vi "Show_Queued_Images.vi"(8 "error in (no error)":errorcluster, 11 "ImagesQueue":string) -> (0 "error out":errorcluster)   [LabVIEW 2016]
uses:
  <vilib>/vision/Image Controls.llb/IMAQ Image.ctl
panel:
  out "Image":T1(plugin-control)
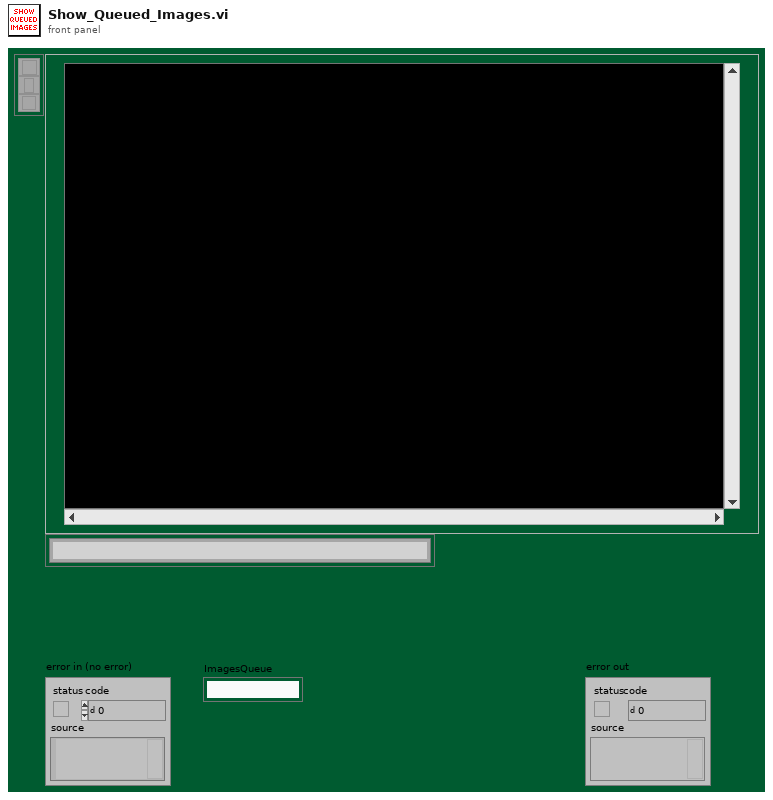
[diagram p1: front panel]
types:
  T1 = typedef "IMAQ Image.ctl" = refnum<image>
  T2 = enum16{"Show:ResetError", "Show:Exit", "Show:QueueError", "Show;Timeout_Image_Queue", "Show:Error_Imaq", "Show:Reset_Error_Recvd"}
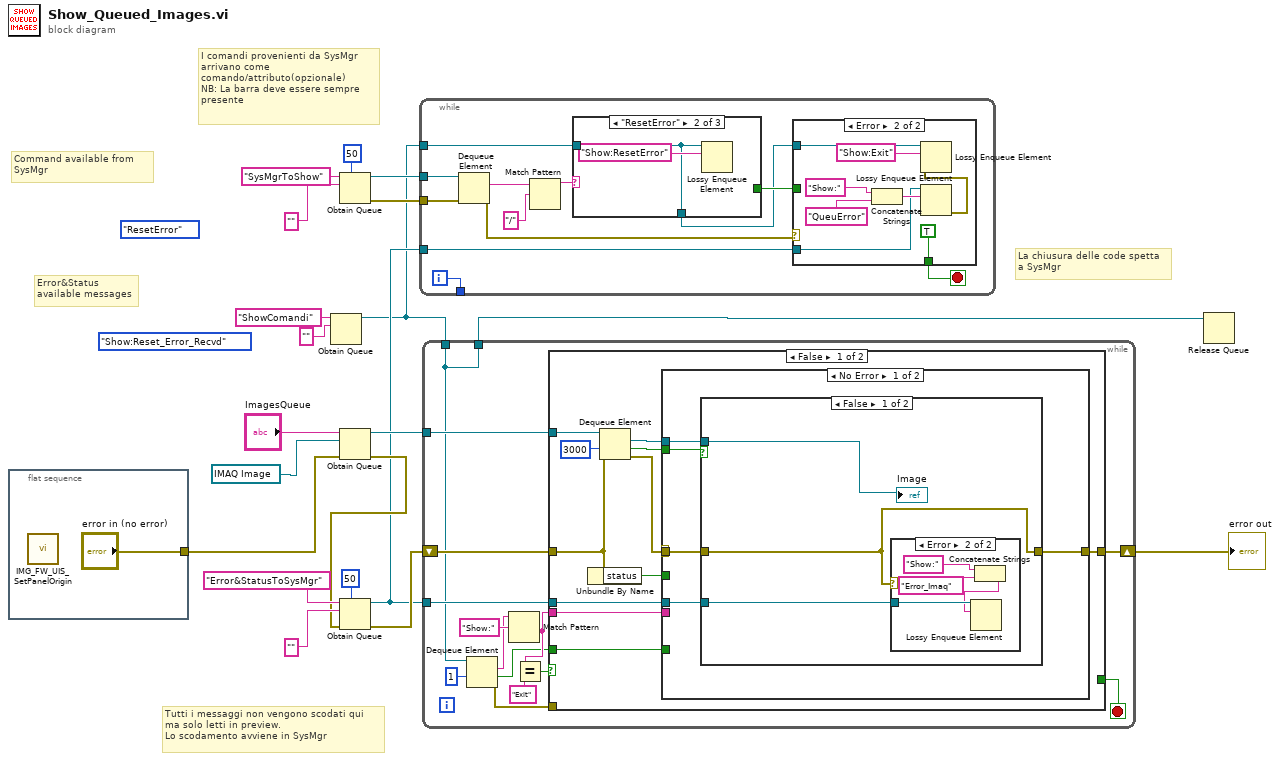
[diagram p0: block diagram]
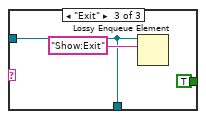
[diagram p4: hidden frame]
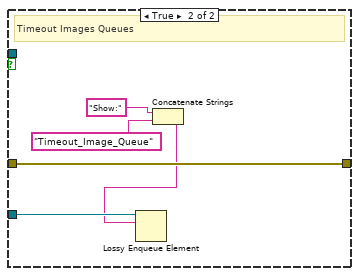
[diagram p6: hidden frame]
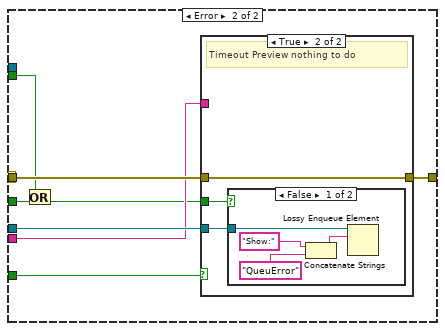
[diagram p7: hidden frame]
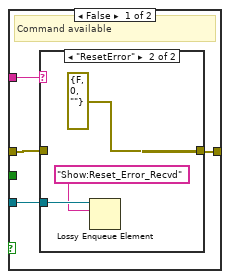
[diagram p8: hidden frame]
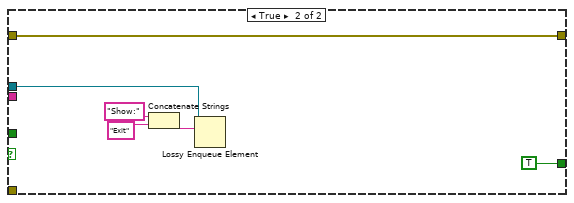
[diagram p11: hidden frame]
diagram:
  (unwired) T2."Show:Reset_Error_Recvd"
  (unwired) enum16{"Exit", "ResetError"}."ResetError"
  # "Tutti i messaggi non vengono scodati qui\nma solo letti in preview.\nLo scodamento avviene in SysMgr"
  # "Error&Status\navailable messages"
  # "Command available from \nSysMgr"
  # "La chiusura delle code spetta\na SysMgr"
  # "I comandi provenienti da SysMgr \narrivano come\ncomando/attributo(opzionale)\nNB: La barra deve essere sempre \npresente"
  n1 = flat-sequence {
    tunnel: ["error in (no error)"] -> w9
    frame #0 {
      n2 = call "IMG_FW_UIS_SetPanelOrigin.vi"() -> ()  [unwired: 11 in, 1 out]
    }
  }
  n3 = Obtain Queue(name (unnamed)="ShowComandi", element data type="") -> (queue out=w3:refnum<queue>)  [unwired: 3 in, 2 out]
  n4 = Obtain Queue(max queue size (-1, unlimited)=50, name (unnamed)="SysMgrToShow", element data type="") -> (queue out=w16:refnum<queue>, error out=w10:errorcluster)  [unwired: 2 in, 1 out]
  n5 = Obtain Queue(name (unnamed)="ImagesQueue", element data type=T1 refnum ("Image"), error in (no error)=w9) -> (queue out=w19:refnum<queue>, error out=w8:errorcluster)  [unwired: 2 in, 1 out]
  n6 = Obtain Queue(max queue size (-1, unlimited)=50, name (unnamed)="Error&StatusToSysMgr", element data type="", error in (no error)=w8) -> (queue out=w4:refnum<queue>, error out=w7:errorcluster)  [unwired: 1 in, 1 out]
  n7 = while {
    tunnel: w16 -> [w33]
    tunnel: w10 -> [w29]
    tunnel: w4 -> [w26]
    tunnel: [w24] -> _
    tunnel: w3 -> [w22]
    i -> [w24]
    stop <- w27 stop-if-true
    n8 = Dequeue Element(queue=w33, error in (no error)=w29) -> (element=w32:string, error out=w28:errorcluster)  [unwired: 1 in, 2 out]
    n9 = Match Pattern(string=w32, regular expression="/") -> (before substring=w30:string)  [unwired: 1 in, 3 out]
    n10 = case shown="\"ResetError\"" w30 {
      tunnel: [w43 w44 w46] -> w23
      tunnel: [_ _ TRUE] -> w25
      tunnel: w22 -> [w43 w44 w46]
      frame "", Default {
      }
      frame "ResetError" {
        n11 = Lossy Enqueue Element(queue=w44, element="Show:ResetError" ("notification")) -> ()  [unwired: 1 in, 4 out]
      }
      frame "Exit" {
        n12 = Lossy Enqueue Element(queue=w46, element="Show:Exit" ("notification")) -> ()  [unwired: 1 in, 4 out]
      }
    }
    n13 = case shown="Error" w28 {
      tunnel: [w34 TRUE] -> w27
      tunnel: w26 -> [_ w38]
      tunnel: w25 -> [w34 _]
      tunnel: w23 -> [_ w35]
      frame No Error {
      }
      frame Error {
        n14 = Concatenate Strings("Show:", "QueuError") -> (w39:string)
        n15 = Lossy Enqueue Element(queue=w38, element=w39) -> (error out=w37:errorcluster)  [unwired: 1 in, 3 out]
        n16 = Lossy Enqueue Element(queue=w35, element="Show:Exit" ("notification"), error in (no error)=w37) -> ()  [unwired: 4 out]
      }
    }
  }
  n17 = while {
    tunnel: w19 -> [w62]
    tunnel: w4 -> [w56]
    shift-right: [w61] -> w18
    shift-left: w7 -> [w60]
    tunnel: w3 -> [w52]
    tunnel: [w52] -> w2
    stop <- w54 stop-if-true
    n18 = Dequeue Element(queue=w52, timeout in ms (-1)=1) -> (element=w51:string, timed out?=w49:bool, error out=w53:errorcluster)  [unwired: 1 in, 1 out]
    n19 = Match Pattern(string=w51, regular expression="Show:") -> (after substring=w50:string)  [unwired: 1 in, 3 out]
    n20 = Equal?(x=w50, y="Exit") -> (x = y?=w55:bool)
    n21 = case shown="False" w55 {
      tunnel: w62 -> [w73 _]
      tunnel: [w71 w119] -> w61
      tunnel: w60 -> [w67 w119]
      tunnel: w56 -> [w65 w115]
      tunnel: [_ TRUE] -> w54
      tunnel: w53 -> [_ _]
      tunnel: w50 -> [w64 _]
      tunnel: w49 -> [w63 _]
      frame False {
        n22 = Unbundle By Name(w67) -> ("status"=w66:bool)
        n23 = Dequeue Element(queue=w73, timeout in ms (-1)=3000, error in (no error)=w67) -> (element=w72:T1, timed out?=w69:bool, error out=w68:errorcluster)  [unwired: 1 out]
        n24 = case shown="No Error" w68 {
          selector: w68 -> [w75 w98]
          tunnel: w72 -> [w78 _]
          tunnel: w68 -> [_ _]
          tunnel: [w77 w97] -> w71
          tunnel: w69 -> [w76 w94]
          tunnel: w65 -> [w74 w96]
          tunnel: w66 -> [_ w95]
          tunnel: w64 -> [_ w93]
          tunnel: w63 -> [_ w91]
          frame No Error {
            n25 = case shown="False" w76 {
              tunnel: w78 -> [w80 _]
              tunnel: w75 -> [w79 w90]
              tunnel: [w79 w90] -> w77
              tunnel: w74 -> [w81 w89]
              frame False {
                n26 = case shown="Error" w79 {
                  tunnel: w81 -> [_ w85]
                  frame No Error {
                  }
                  frame Error {
                    n27 = Concatenate Strings("Show:", "Error_Imaq") -> (w83:string)
                    n28 = Lossy Enqueue Element(queue=w85, element=w83) -> ()  [unwired: 1 in, 4 out]
                  }
                }
                "Image" <- w80
              }
              frame True {
                # "Timeout Images Queues"
                n29 = Concatenate Strings("Show:", "Timeout_Image_Queue" ("string")) -> (w87:string)
                n30 = Lossy Enqueue Element(queue=w89, element=w87) -> ()  [unwired: 1 in, 4 out]
              }
            }
          }
          frame Error {
            n31 = Or(x=w94, y=w95) -> (x .or. y?=w92:bool)
            n32 = case shown="True" w91 {
              tunnel: [w100 w109] -> w97
              tunnel: w98 -> [w101 w109]
              tunnel: w93 -> [w102 _]
              tunnel: w96 -> [w99 w108]
              tunnel: w92 -> [_ w107]
              frame False {
                # "Command available"
                n33 = case shown="\"ResetError\"" w102 {
                  tunnel: w101 -> [w103 _]
                  tunnel: [w103 errorcluster {"status"=FALSE, "code"=0, "source"=""} ("error constant")] -> w100
                  tunnel: w99 -> [_ w105]
                  frame "False", Default {
                  }
                  frame "ResetError" {
                    n34 = Lossy Enqueue Element(queue=w105, element="Show:Reset_Error_Recvd") -> ()  [unwired: 1 in, 4 out]
                  }
                }
              }
              frame True {
                # "Timeout Preview nothing to do"
                n35 = case shown="False" w107 {
                  tunnel: w108 -> [w113 _]
                  frame False {
                    n36 = Concatenate Strings("Show:", "QueuError") -> (w110:string)
                    n37 = Lossy Enqueue Element(queue=w113, element=w110) -> ()  [unwired: 1 in, 4 out]
                  }
                  frame True {
                  }
                }
              }
            }
          }
        }
      }
      frame True {
        n38 = Concatenate Strings("Show:", "Exit") -> (w117:string)
        n39 = Lossy Enqueue Element(queue=w115, element=w117) -> ()  [unwired: 1 in, 4 out]
      }
    }
  }
  "error out" <- w18
  n40 = Release Queue(queue=w2) -> ()  [unwired: 2 in, 3 out]
